vi "Find Center.vi"(7 "Tray Number":dbl format="%#_13g", 9 "XYZTheta":dbl[](array[numeric]), 10 "Motion.lvclass":refnum<class "Motion.lvclass">) -> (1 "XYZTheta Centers":dbl[][](array[numeric])=[[878.4985063746162, 239.94637460510748, 54.08724761972906, -3.1387193230847177], [988.4985063746162, 209.94637460510748, 54.08724761972906, 0.0]], 2 "Motion Out":refnum<class "Motion.lvclass">)   [LabVIEW 2016, in "Assembly Tray.lvclass"]
uses:
  Assembly Tray.lvclass
  Find Tray.ctl
  Controller/Motion/Motion.lvclass
  Controller/Motion/A3200/A3200.lvclass
  Controller/Camera/Machine Vision.ctl
  Controller/Camera/Camera.lvclass
panel:
  in  "Speed XY":dbl=5.0
  in  "Jog Cluster":T1={"Jog XY Cluster"={"object goes up"=FALSE, "object goes down"=FALSE, "object goes right"=FALSE, "object goes left"=FALSE, "SW2"=FALSE, "SW1"=FALSE, "YY (mm)"=0.1, "YN (mm) "=0.01, "NY (mm) "=0.005, "NN (mm) "=0.001}, "Jog Z Cluster "={"Z go down 0.1 mm"=FALSE, "Z go up 0.1 mm"=FALSE, "Z go down 0.05 mm"=FALSE, "Z go up 0.05 mm"=FALSE, "Z go down 0.01 mm"=FALSE, "Z go up 0.01 mm"=FALSE, "Z go down"=FALSE, "Z go up"=FALSE, "step (mm)"=0.001}}
  in  "Change light":bool
  in  "light":dbl=5.0
  in  "Machine Vision 2":T2
  out "Image 2":T3(plugin-control)
  in  "XY Go Sum":bool
  in  "Machine Vision":T2
  out "Right Fiducial":dbl[](array[numeric])=[833.8468401167813, 156.2705176060632, 54.03258858141665]
  out "Left Fiducial":dbl[](array[numeric])=[923.150172632451, 323.62223160415175, 54.14190665804148]
  out "Gantry":dbl[](array[numeric])=[833.8468482802334, 156.27047808579954, 54.03258861193423, 2.7274344405293465]
  out "Sum":dbl[](array[numeric])
  out "Camera":dbl[](array[numeric])
  in  "Carrier Tray":T4
  out "Image":T3(plugin-control)
  out "Center":dbl[](array[numeric])=[878.4985063746162, 239.94637460510748, 54.08724761972906, -3.1387193230847177]
  in  "Position Number":i16=1
  in  "Go to Center":bool
  in  "Calculate":bool
  in  "Record Bottom":bool
  in  "Record Top":bool
  in  "Go to Bottom Fiducial":bool
  in  "Go to Top Fiducial":bool
  in  "Joystick":bool
  in  "Stop":bool
  # "1"
  # "2"
  # "Light \nAcrylic : 5"
  # "Machine Vision:\nAcrylic : None"
  # "position 1"
  # "position 2"
  # "Acrylic Baseplate"
  # "3"
  # "Baseplate alignment 定位底板"
  # "1. 選擇視覺辨識\n2. 選擇亮度\n3. Go To Top Fiducial到第一定位點，點選Joystick進行定位\n4. Record Top 紀錄第一點\n5. Go To Bottom Fiducial 到第二定位點，點選Joystick進行定位\n6. Record Bottom 紀錄第二點\n7. Go to Center 到中心點 檢查是否定位結果正常\n8. Submit 結束baseplate定位"
  # "4"
  # "5"
  # "6"
  # "7"
  # "8"
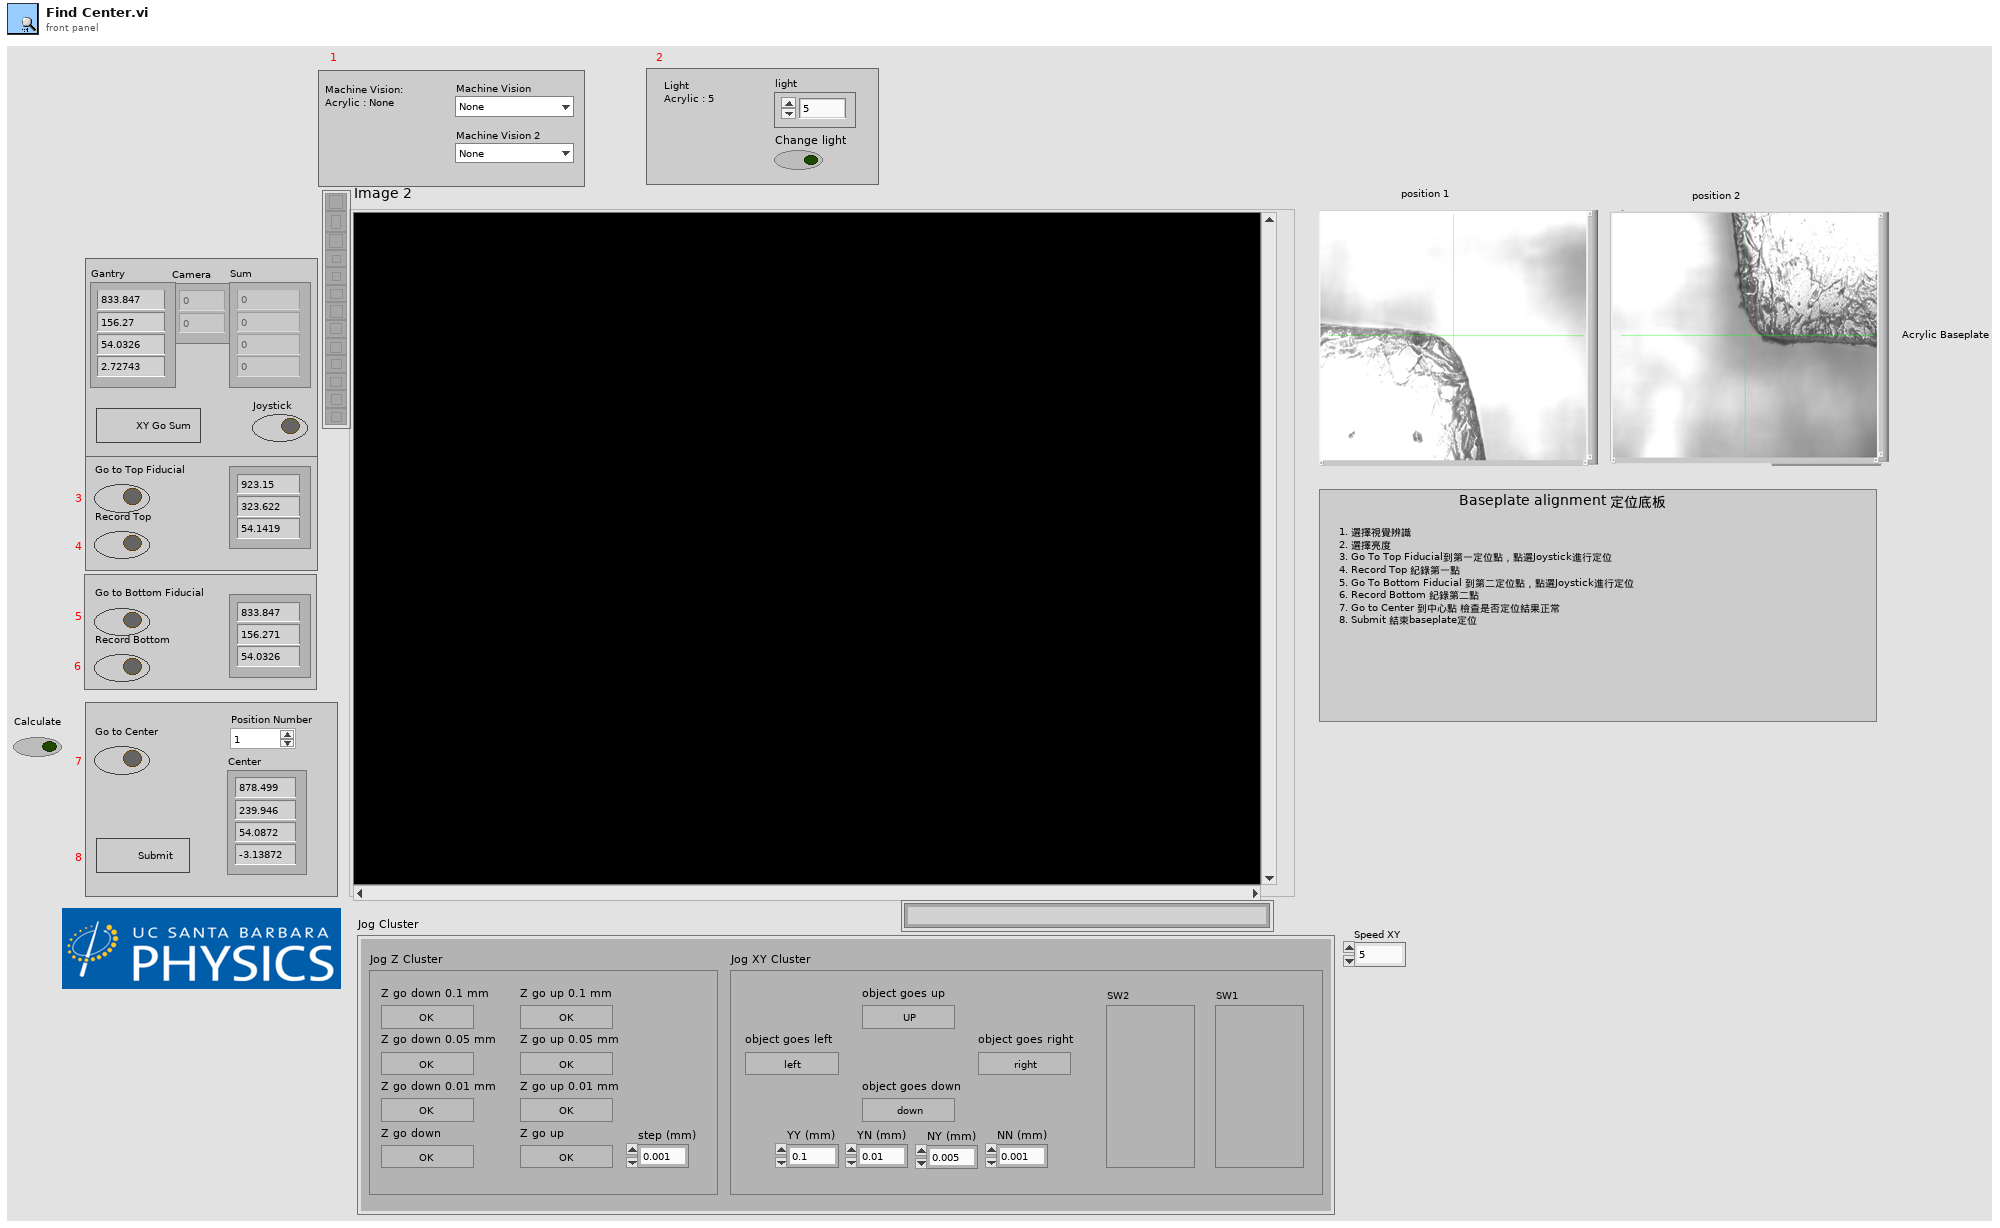
[diagram p1: front panel]
types:
  T1 = cluster{"Jog XY Cluster":cluster{"object goes up":bool, "object goes down":bool, "object goes right":bool, "object goes left":bool, "SW2":bool, "SW1":bool, "YY (mm)":dbl, "YN (mm) ":dbl, "NY (mm) ":dbl, "NN (mm) ":dbl}, "Jog Z Cluster ":cluster{"Z go down 0.1 mm":bool, "Z go up 0.1 mm":bool, "Z go down 0.05 mm":bool, "Z go up 0.05 mm":bool, "Z go down 0.01 mm":bool, "Z go up 0.01 mm":bool, "Z go down":bool, "Z go up":bool, "step (mm)":dbl}}
  T2 = typedef "Camera.lvclass/Machine Vision.ctl" = enum16{"None", "Circle", "Tray Fiducials", "Tray Fiducials, top right", "HPK Silicon square", "HPK Silicon", "8inch PCB Pad", "Hexaboard", "Corner (TL, BR)", "Corner (BL, TR)"}
  T3 = typedef "IMAQ Image.ctl" = refnum<image>
  T4 = typedef "Assembly Tray.lvclass/Find Tray.ctl" = cluster{"Gantry Fiducials":dbl[], "Relative Coordinates":dbl[][], "Camera Fiducials":dbl[][], "XYZTheta Centers":dbl[][], "Workspace Center":dbl[], "Syringe Relative Coordinates":dbl[], "Gantry Region":dbl, "Fiducials":path}
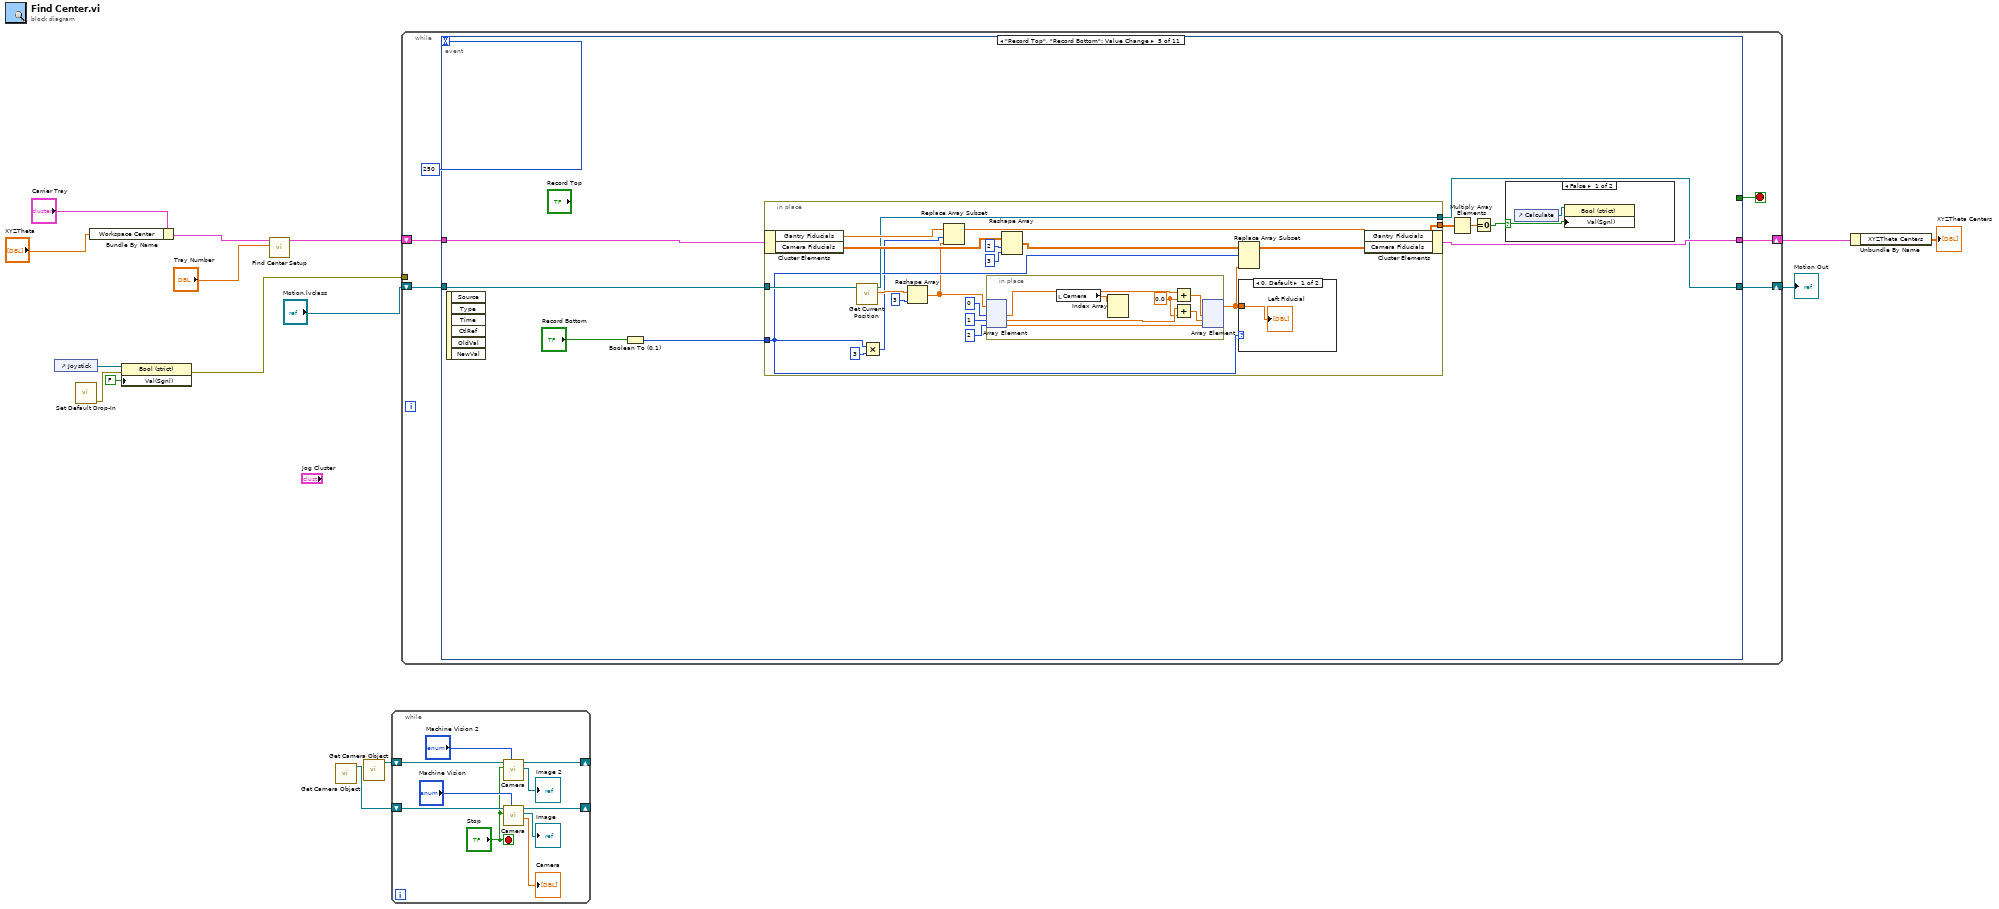
[diagram p0: block diagram]
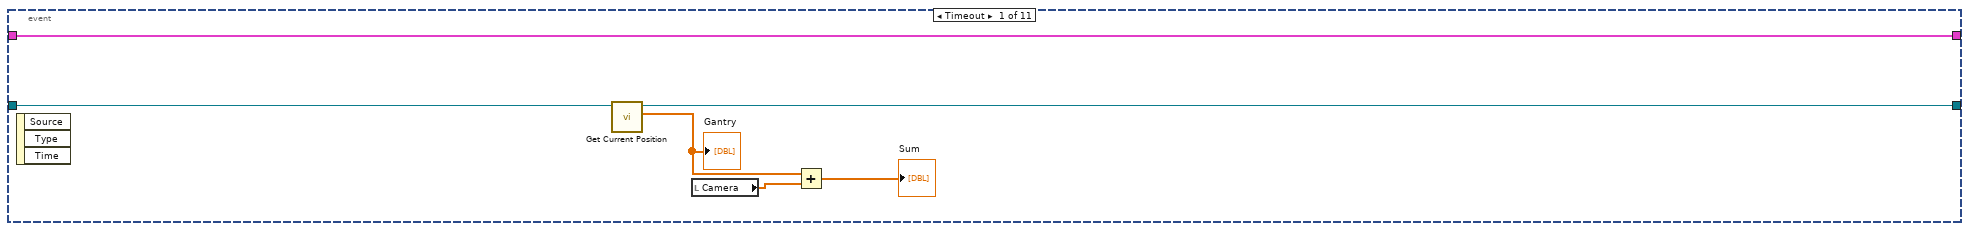
[diagram p2: hidden frame]
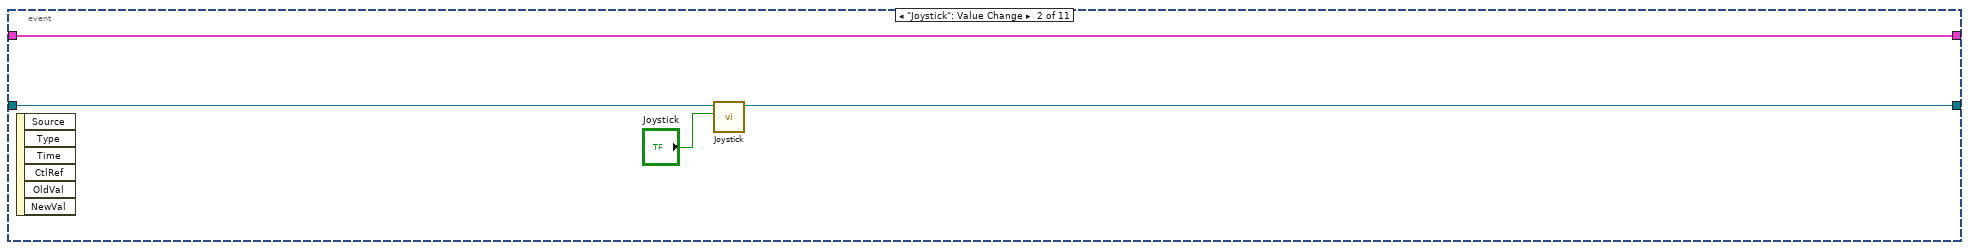
[diagram p3: hidden frame]
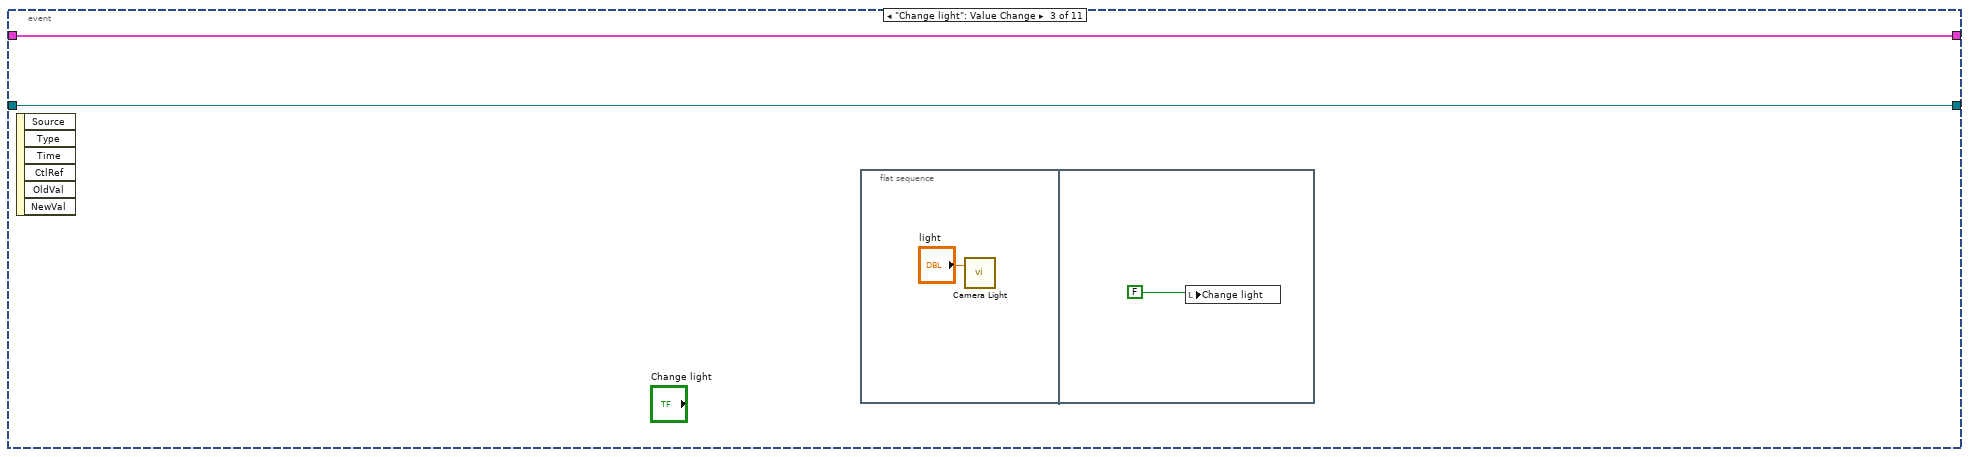
[diagram p4: hidden frame]
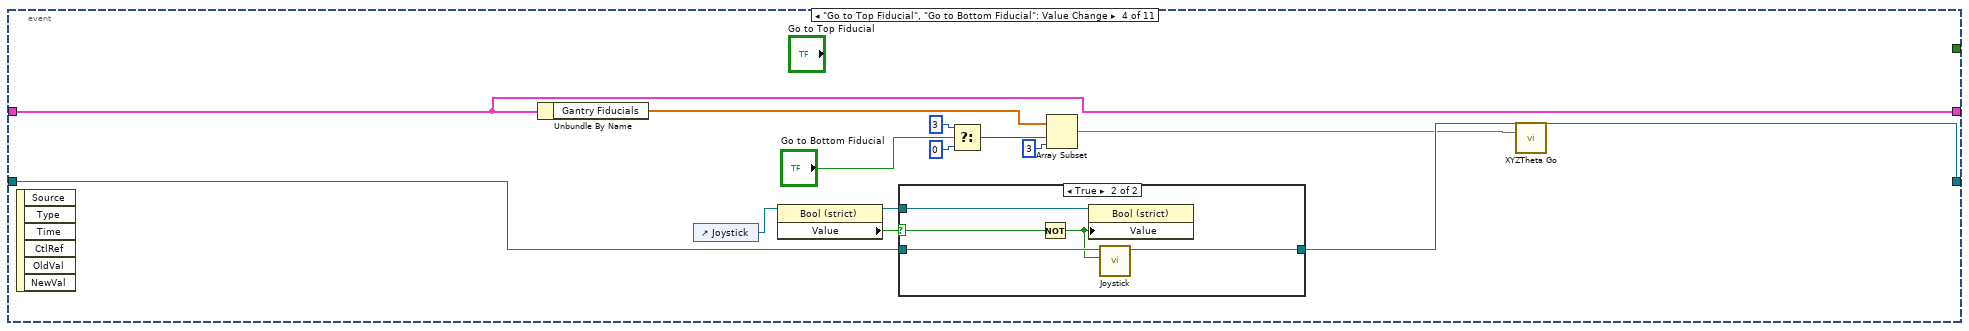
[diagram p5: hidden frame]
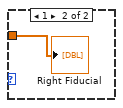
[diagram p8: hidden frame]
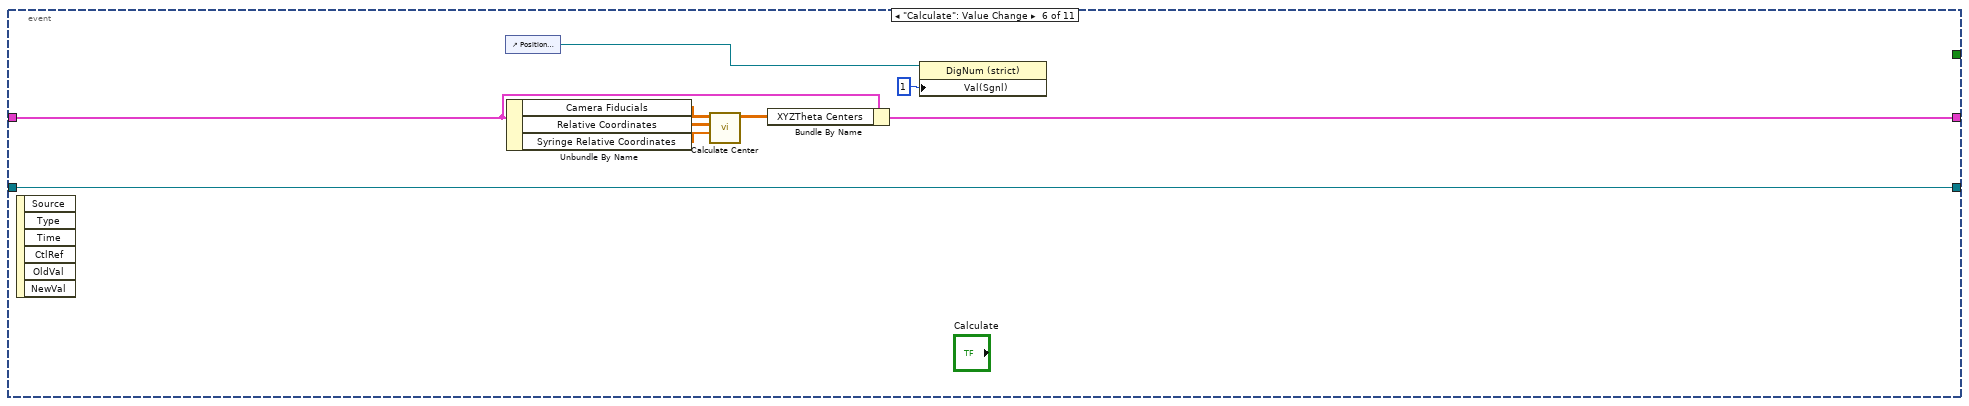
[diagram p9: hidden frame]
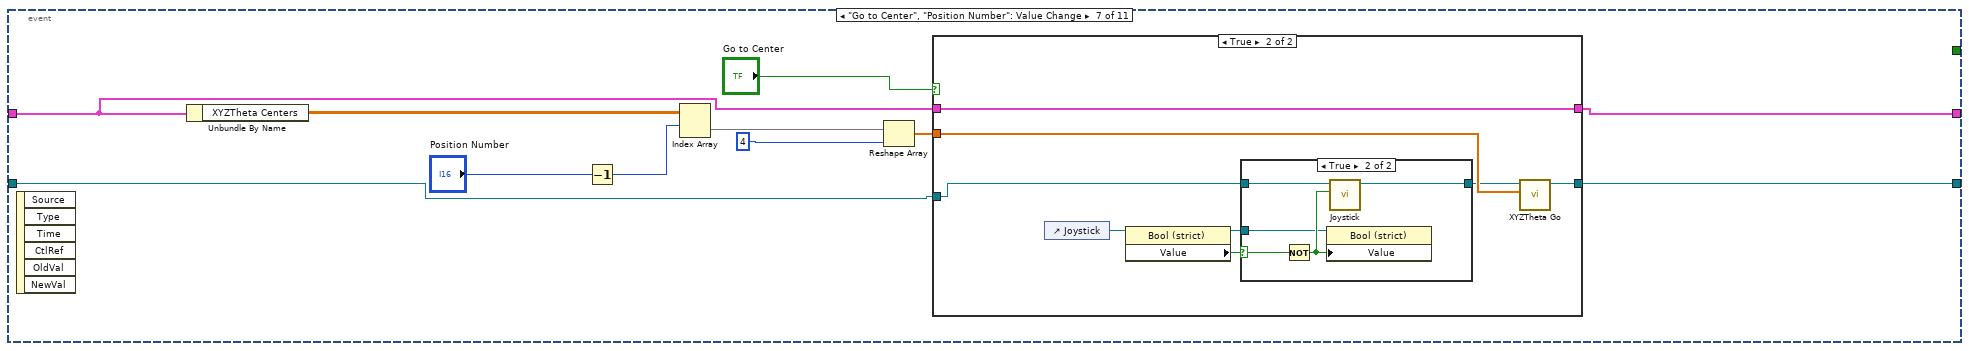
[diagram p10: hidden frame]
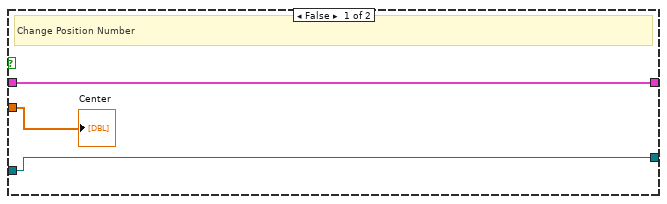
[diagram p11: hidden frame]
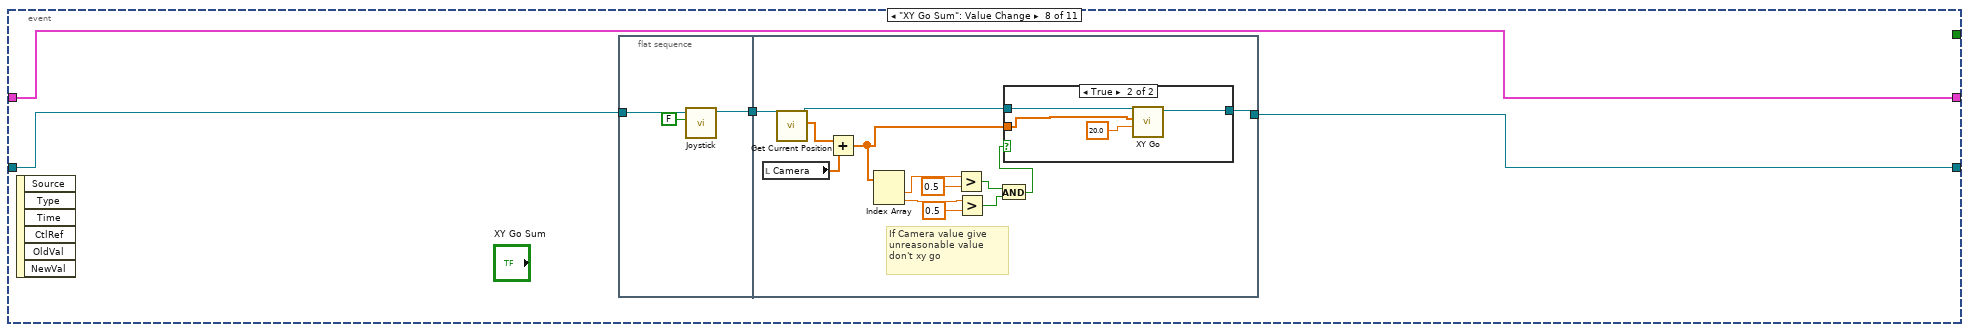
[diagram p13: hidden frame]
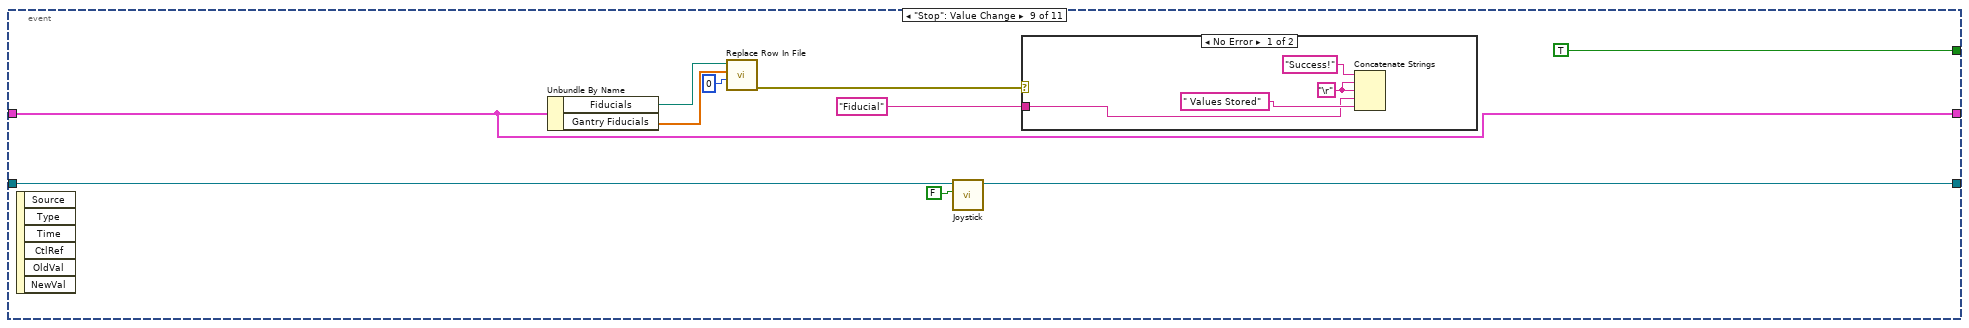
[diagram p15: hidden frame]
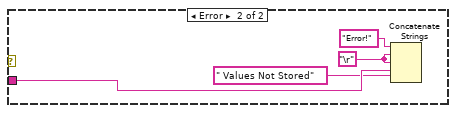
[diagram p16: hidden frame]
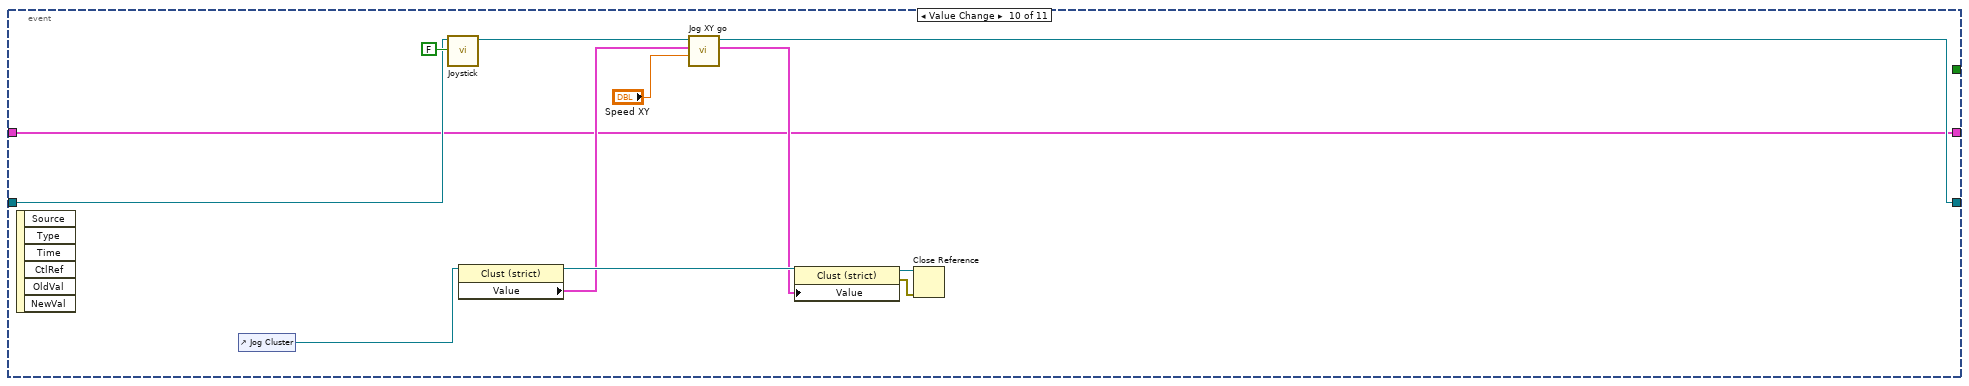
[diagram p17: hidden frame]
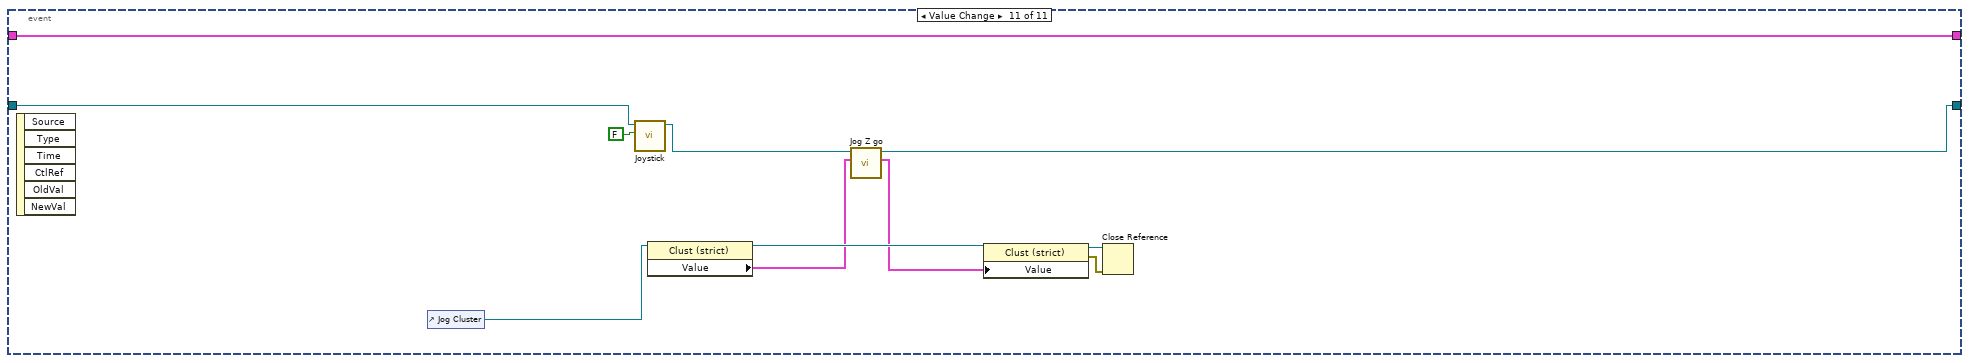
[diagram p18: hidden frame]
diagram:
  n1 = control-ref of="Joystick"() -> (w15:refnum<vi>)
  n2 = call "Set Default Drop-In.vi"() -> ("error out"=w7:errorcluster)  [unwired: 11 in]
  n3 = Bundle By Name(cluster="Carrier Tray", "Workspace Center"="XYZTheta") -> (w9:T4)
  n4 = property class="Bool (strict)"(reference=w15, error in=w7, "Val(Sgnl)"=FALSE) -> (error out=w13:errorcluster)  [unwired: 1 out]
  n5 = call "Find Center Setup.vi"("Carrier Tray"=w9, "Tray Number"="Tray Number") -> ("Assembly Tray Out"=w12:T4)  [unwired: 8 in]
  n6 = call "Get Camera Object.vi"() -> ("Camera out"=w2:refnum<class "Camera.lvclass">)  [unwired: 10 in, 1 out]
  n7 = call "Get Camera Object.vi"() -> ("Camera out"=w1:refnum<class "Camera.lvclass">)  [unwired: 10 in, 1 out]
  n8 = while {
    shift-right: [w21] -> _
    shift-left: w2 -> [w25]
    shift-right: [w19] -> _
    shift-left: w1 -> [w20]
    stop <- "Stop" stop-if-true
    n9 = call "Camera.vi"("Machine Vision"="Machine Vision 2", "Stop"="Stop", "Camera in"=w20) -> ("Image"=→"Image 2":T3, "Camera out"=w19:refnum<class "Camera.lvclass">)  [unwired: 5 in, 2 out]
    n10 = call "Camera.vi"("Machine Vision"="Machine Vision", "Stop"="Stop", "Camera in"=w25) -> ("Camera"=→"Camera":dbl[], "Image"=→"Image":T3, "Camera out"=w21:refnum<class "Camera.lvclass">)  [unwired: 5 in, 1 out]
  }
  n11 = while {
    shift-right: [w30] -> w11
    shift-left: w12 -> [w31]
    tunnel: w13 -> [_]
    shift-right: [w26] -> w4
    shift-left: "Motion.lvclass" -> [w27]
    stop <- w29 stop-if-true
    n12 = event shown="[4] \"Record Top\", \"Record Bottom\": Value Change" {
      selector: _ -> [_ _ _ _ _ _ _ _ _ _ _]
      dyn-events: _ -> [_ _ _ _ _ _ _ _ _ _ _]
      timeout: 250 -> [_ _ _ _ _ _ _ _ _ _ _]
      tunnel: [w33 w39 w42 w59 w74 w107 w120 w142 w170 w185 w197] -> w30
      tunnel: w31 -> [w33 w39 w42 w59 w68 w111 w121 w142 w170 w185 w197]
      tunnel: [_ _ _ _ _ _ _ _ TRUE _ _] -> w29
      tunnel: w27 -> [w34 w40 w43 w50 w67 w105 w118 w145 w172 w188 w200]
      tunnel: [w32 w38 w43 w46 w66 w105 w117 w143 w171 w186 w199] -> w26
      event Timeout {
        n13 = event-data() -> ()  [unwired: 1 in, 3 out]
        n14 = call-dynamic "Get Current Position.vi"("Motion in"=w34) -> ("XYZTheta Out"=w35:dbl[], "Motion out"=w32:refnum<class "Motion.lvclass">)  [unwired: 8 in, 1 out]
        "Gantry" <- w35
        n15 = local read "Camera"() -> (w37:dbl[])
        n16 = Add(x=w35, y=w37) -> (x+y=→"Sum":dbl[])
      }
      event "Joystick": Value Change {
        n17 = event-data() -> ()  [unwired: 1 in, 6 out]
        n18 = call-dynamic "Joystick.vi"("Joystick"="Joystick", "Motion in"=w40) -> ("Motion out"=w38:refnum<class "Motion.lvclass">)  [unwired: 8 in, 1 out]
      }
      event "Change light": Value Change {
        n19 = event-data() -> ()  [unwired: 1 in, 6 out]
        n20 = flat-sequence {
          frame #0 {
            n21 = call "Camera Light.vi"("input"="light") -> ()  [unwired: 2 in, 1 out]
          }
          frame #1 {
            n22 = local write "Change light"(FALSE) -> ()
          }
        }
      }
      event "Go to Top Fiducial", "Go to Bottom Fiducial": Value Change {
        n23 = event-data() -> ()  [unwired: 1 in, 6 out]
        n24 = Unbundle By Name(w59) -> ("Gantry Fiducials"=w57:dbl[])
        n25 = control-ref of="Joystick"() -> (w58:refnum<vi>)
        n26 = property class="Bool (strict)"(reference=w58) -> (reference out=w49:refnum<vi>, "Value"=w51:bool)  [unwired: 1 in, 1 out]
        n27 = case shown="True" w51 {
          selector: w51 -> [_ w65]
          tunnel: w50 -> [w60 w64]
          tunnel: [w60 w63] -> w48
          tunnel: w49 -> [_ w61]
          frame False {
          }
          frame True {
            n28 = Not(x=w65) -> (.not. x?=w62:bool)
            n29 = property class="Bool (strict)"(reference=w61, "Value"=w62) -> ()  [unwired: 1 in, 2 out]
            n30 = call-dynamic "Joystick.vi"("Joystick"=w62, "Motion in"=w64) -> ("Motion out"=w63:refnum<class "Motion.lvclass">)  [unwired: 8 in, 1 out]
          }
        }
        n31 = Select(t=3, s="Go to Bottom Fiducial", f=0) -> (s? t:f=w55:i32)
        n32 = Array Subset(array=w57, index=w55, length=3) -> (w47:dbl[])
        n33 = call "XYZTheta Go.vi"("XYZTheta In"=w47, "Motion in"=w48) -> ("Motion out"=w46:refnum<class "Motion.lvclass">)  [unwired: 7 in, 2 out]
      }
      event "Record Top", "Record Bottom": Value Change {
        n34 = event-data() -> ()  [unwired: 1 in, 6 out]
        n35 = Boolean To (0,1)(Boolean="Record Bottom") -> (0, 1=w70:i16)
        n36 = in-place {
          in-place-border: [w89] -> w71
          in-place-border: w70 -> [w82]
          in-place-border: w67 -> [w84]
          in-place-border: [w83] -> w66
          n37 = in-place-cluster #1(w68) -> ("Gantry Fiducials"=w86:dbl[], "Camera Fiducials"=w93:dbl[][])
          n38 = call-dynamic "Get Current Position.vi"("Motion in"=w84) -> ("XYZTheta Out"=w87:dbl[], "Motion out"=w83:refnum<class "Motion.lvclass">)  [unwired: 8 in, 1 out]
          n39 = Multiply(x=w82, y=i16 3) -> (x*y=w80:i16)
          n40 = Reshape Array(w87, 3 ("dimension size")) -> (w79:dbl[])
          n41 = Replace Array Subset(array=w86, new element=w79, index=w80) -> (w85:dbl[])
          n42 = in-place {
            w96 = 0.0 ("y")
            n43 = in-place-array #2(w79, 0, 1, 2) -> (w102:dbl, w101:dbl, w98:dbl)
            n44 = local read "Camera"() -> (w97:dbl[])
            n45 = Index Array(array=w97) -> ()  [unwired: 2 in, 2 out]
            n46 = Add(x=w102, y=w96) -> (x+y=w99:dbl)
            n47 = Add(x=w101, y=w96) -> (x+y=w100:dbl)
            n48 = in-place-array #2(w99, w100, w98) -> (w78:dbl[])  [unwired: 3 out]
          }
          n49 = Reshape Array(w93, 2 ("length"), 3 ("dimension size")) -> (w92:dbl[][])
          n50 = Replace Array Subset(array=w92, new element=w78, index (row)=w82) -> (w89:dbl[][])  [unwired: 1 in]
          n51 = case shown="0, Default" w82 {
            tunnel: w78 -> [w103 w104]
            frame 0, Default {
              "Left Fiducial" <- w103
            }
            frame 1 {
              "Right Fiducial" <- w104
            }
          }
          n52 = in-place-cluster #1("Gantry Fiducials"=w85, "Camera Fiducials"=w89) -> (w74:T4)
        }
        n53 = Multiply Array Elements(1:w71) -> (0:w73:dbl)
        n54 = Equal To 0?(x=w73) -> (x = 0?=w72:bool)
        n55 = case shown="False" w72 {
          selector: w72 -> [w75 _]
          frame False {
            n56 = control-ref of="Calculate"() -> (w76:refnum<vi>)
            n57 = property class="Bool (strict)"(reference=w76, "Val(Sgnl)"=w75) -> ()  [unwired: 1 in, 2 out]
          }
          frame True {
          }
        }
      }
      event "Calculate": Value Change {
        n58 = event-data() -> ()  [unwired: 1 in, 6 out]
        n59 = control-ref of="Position Number"() -> (w113:refnum<vi>)
        n60 = Unbundle By Name(w111) -> ("Camera Fiducials"=w110:dbl[][], "Relative Coordinates"=w109:dbl[][], "Syringe Relative Coordinates"=w106:dbl[])
        n61 = call "Calculate Center.vi"("Syringe Coordinates"=w106, "Relative Coordinates"=w109, "Fiducial Measurements"=w110) -> ("XYZTheta Centers"=w108:dbl[][])  [unwired: 8 in]
        n62 = Bundle By Name(cluster=w111, "XYZTheta Centers"=w108) -> (w107:T4)
        n63 = property class="DigNum (strict)"(reference=w113, "Val(Sgnl)"=i16 1 ("Value (Signaling)")) -> ()  [unwired: 1 in, 2 out]
      }
      event "Go to Center", "Position Number": Value Change {
        n64 = event-data() -> ()  [unwired: 1 in, 6 out]
        n65 = Unbundle By Name(w121) -> ("XYZTheta Centers"=w124:dbl[][])
        n66 = Decrement(x="Position Number") -> (x-1=w122:i16)
        n67 = Index Array(array=w124, index (row)=w122) -> (element=w115:dbl[])  [unwired: 1 in]
        n68 = Reshape Array(w115, u32 4) -> (w114:dbl[])
        n69 = case shown="True" "Go to Center" {
          tunnel: w114 -> [w127 w133]
          tunnel: w121 -> [w126 w135]
          tunnel: [w126 w135] -> w120
          tunnel: w118 -> [w125 w129]
          tunnel: [w125 w134] -> w117
          frame False {
            # "Change Position Number"
            "Center" <- w127
          }
          frame True {
            n70 = control-ref of="Joystick"() -> (w132:refnum<vi>)
            n71 = property class="Bool (strict)"(reference=w132) -> (reference out=w130:refnum<vi>, "Value"=w131:bool)  [unwired: 1 in, 1 out]
            n72 = case shown="True" w131 {
              selector: w131 -> [_ w141]
              tunnel: w129 -> [w136 w140]
              tunnel: [w136 w139] -> w128
              tunnel: w130 -> [_ w137]
              frame False {
              }
              frame True {
                n73 = Not(x=w141) -> (.not. x?=w138:bool)
                n74 = property class="Bool (strict)"(reference=w137, "Value"=w138) -> ()  [unwired: 1 in, 2 out]
                n75 = call-dynamic "Joystick.vi"("Joystick"=w138, "Motion in"=w140) -> ("Motion out"=w139:refnum<class "Motion.lvclass">)  [unwired: 8 in, 1 out]
              }
            }
            n76 = call "XYZTheta Go.vi"("XYZTheta In"=w133, "Motion in"=w128) -> ("Motion out"=w134:refnum<class "Motion.lvclass">)  [unwired: 7 in, 2 out]
          }
        }
      }
      event "XY Go Sum": Value Change {
        n77 = event-data() -> ()  [unwired: 1 in, 6 out]
        n78 = flat-sequence {
          tunnel: w145 -> [w148]
          tunnel: [w146] -> w144
          tunnel: w144 -> [w154]
          tunnel: [w161] -> w143
          frame #0 {
            n79 = call-dynamic "Joystick.vi"("Joystick"=FALSE, "Motion in"=w148) -> ("Motion out"=w146:refnum<class "Motion.lvclass">)  [unwired: 8 in, 1 out]
          }
          frame #1 {
            # "If Camera value give unreasonable value \ndon't xy go"
            n80 = local read "Camera"() -> (w151:dbl[])
            n81 = call-dynamic "Get Current Position.vi"("Motion in"=w154) -> ("XYZTheta Out"=w152:dbl[], "Motion out"=w153:refnum<class "Motion.lvclass">)  [unwired: 8 in, 1 out]
            n82 = Add(x=w152, y=w151) -> (x+y=w150:dbl[])
            n83 = Index Array(array=w150) -> (element #1=w160:dbl, element #2=w158:dbl)  [unwired: 2 in]
            n84 = Greater?(x=w160, y=0.5) -> (0:w156:bool)
            n85 = Greater?(x=w158, y=0.5) -> (0:w155:bool)
            n86 = And(x=w156, y=w155) -> (x .and. y?=w149:bool)
            n87 = case shown="True" w149 {
              tunnel: w153 -> [w162 w166]
              tunnel: [w162 w165] -> w161
              tunnel: w150 -> [_ w163]
              frame False {
              }
              frame True {
                n88 = call-dynamic "XY Go.vi"("Speed"=20.0, "XY"=w163, "Motion in"=w166) -> ("Motion out"=w165:refnum<class "Motion.lvclass">)  [unwired: 7 in, 1 out]
              }
            }
          }
        }
      }
      event "Stop": Value Change {
        n89 = event-data() -> ()  [unwired: 1 in, 6 out]
        n90 = Unbundle By Name(w170) -> ("Fiducials"=w168:path, "Gantry Fiducials"=w169:dbl[])
        n91 = call "Replace Row In File.vi"("Index"=0, "Insert Array"=w169, "Path"=w168) -> ("error out"=w175:errorcluster)  [unwired: 8 in]
        n92 = call-dynamic "Joystick.vi"("Joystick"=FALSE, "Motion in"=w172) -> ("Motion out"=w171:refnum<class "Motion.lvclass">)  [unwired: 8 in, 1 out]
        n93 = case shown="No Error" w175 {
          tunnel: "Fiducial" -> [w177 w184]
          frame No Error {
            w178 = "\r"
            n94 = Concatenate Strings("Success!", w178, w178, w177, " Values Stored") -> ()  [unwired: 1 out]
          }
          frame Error {
            w181 = "\r"
            n95 = Concatenate Strings("Error!", w181, w181, w184, " Values Not Stored") -> ()  [unwired: 1 out]
          }
        }
      }
      event "Jog Cluster.Jog XY Cluster.object goes up", "Jog Cluster.Jog XY Cluster.object goes down", "Jog Cluster.Jog XY Cluster.object goes right", "Jog Cluster.Jog XY Cluster.object goes left": Value Change {
        n96 = event-data() -> ()  [unwired: 1 in, 6 out]
        n97 = control-ref of="Jog Cluster"() -> (w189:refnum<vi>)
        n98 = call-dynamic "Joystick.vi"("Joystick"=FALSE, "Motion in"=w188) -> ("Motion out"=w187:refnum<class "Motion.lvclass">)  [unwired: 8 in, 1 out]
        n99 = property class="Clust (strict)"(reference=w189) -> (reference out=w194:refnum<vi>, "Value"=w191:T1)  [unwired: 1 in, 1 out]
        n100 = call "Jog XY go.vi"("Speed"="Speed XY", "Jog Cluster IN"=w191, "Motion.lvclass IN"=w187) -> ("Jog Cluster OUT"=w190:T1, "Motion.lvclass OUT"=w186:refnum<class "Motion.lvclass">)  [unwired: 7 in]
        n101 = property class="Clust (strict)"(reference=w194, "Value"=w190) -> (reference out=w192:refnum<vi>, error out=w193:errorcluster)  [unwired: 1 in]
        n102 = Close Reference(reference=w192, error in (no error)=w193) -> ()  [unwired: 1 out]
      }
      event "Jog Cluster.Jog Z Cluster.Z go down 0.1 mm", "Jog Cluster.Jog Z Cluster.Z go up 0.1 mm", "Jog Cluster.Jog Z Cluster.Z go down 0.05 mm", "Jog Cluster.Jog Z Cluster.Z go up 0.05 mm", "Jog Cluster.Jog Z Cluster.Z go down 0.01 mm", "Jog Cluster.Jog Z Cluster.Z go up 0.01 mm", "Jog Cluster.Jog Z Cluster.Z go down", "Jog Cluster.Jog Z Cluster.Z go up": Value Change {
        n103 = event-data() -> ()  [unwired: 1 in, 6 out]
        n104 = control-ref of="Jog Cluster"() -> (w204:refnum<vi>)
        n105 = call-dynamic "Joystick.vi"("Joystick"=FALSE, "Motion in"=w200) -> ("Motion out"=w198:refnum<class "Motion.lvclass">)  [unwired: 8 in, 1 out]
        n106 = property class="Clust (strict)"(reference=w204) -> (reference out=w207:refnum<vi>, "Value"=w202:T1)  [unwired: 1 in, 1 out]
        n107 = call "Jog Z go.vi"("Jog Cluster IN"=w202, "Motion.lvclass IN"=w198) -> ("Jog Cluster OUT"=w201:T1, "Motion.lvclass OUT"=w199:refnum<class "Motion.lvclass">)  [unwired: 8 in]
        n108 = property class="Clust (strict)"(reference=w207, "Value"=w201) -> (reference out=w205:refnum<vi>, error out=w206:errorcluster)  [unwired: 1 in]
        n109 = Close Reference(reference=w205, error in (no error)=w206) -> ()  [unwired: 1 out]
      }
    }
  }
  "Motion Out" <- w4
  n110 = Unbundle By Name(w11) -> ("XYZTheta Centers"=→"XYZTheta Centers":dbl[][])
